vi "Controle_Manip_Main_GUI_WorkingBackup_211222.vi"() -> ()   [LabVIEW 2019] (continued)
                                frame #0 {
                                n1997 = property on="CCD 2D Image Main" class="IntGraph (strict)"("Visible"=FALSE) -> ()  [unwired: 2 in, 2 out]
                                n1998 = property on="CCD 1D Spectrum Main" class="XYGraph (strict)"("Visible"=TRUE) -> ()  [unwired: 2 in, 2 out]
                                }
                                frame #1 {
                                n1999 = local read "Wavelength calibration"() -> (w2451:dbl[])
                                n2000 = local read "CCD ROI"() -> (w2447:T20)
                                n2001 = Divide(x=1239.842, y=w2451) -> (x/y=w2449:dbl[])
                                n2002 = call "PrepareData4Graph.vi"("Wavelength nm"=w2449, "DataLF"=w2454, "CCD ROI"=w2447, "AcqMode"=w2452, "Data type"=T30."Spectre") -> ("Spectrum"=w2453:cluster{"Array 2":dbl[], "Array":dbl[]}, "PLInt out"=w2446:dbl[])  [unwired: 2 in, 2 out]
                                n2003 = local write "CCD 1D Spectrum Main"(w2453) -> ()
                                n2004 = local write "BackgroundSpec"(w2446) -> ()
                                }
                                frame #2 {
                                n2005 = local read "BackgroundSpec"() -> (w2455:dbl[])
                                n2006 = call-poly <vilib>:"Mean.vi"("X"=w2455) -> ("mean"=w2457:dbl)  [unwired: 1 out]
                                n2007 = Negate(x=w2457) -> (-x=w2456:dbl)
                                n2008 = property on="CCD 1D Spectrum Main" class="XYGraph (strict)"("YScale.Offset"=w2456) -> ()  [unwired: 2 in, 2 out]
                                }
                                frame #3 {
                                n2009 = local write "Background taken?"(TRUE ("Background taken?")) -> ()
                                n2010 = property on="Background substract" class="Enum (strict)"("Value"=enum16{"None", "Shutter"}."None" ("Background substract")) -> ()  [unwired: 2 in, 2 out]
                                }
                                }
                                }
                                frame "Image" {
                                n2011 = stacked-sequence {
                                tunnel: w2461 -> [_ w2469]
                                tunnel: w2460 -> [_ w2467]
                                frame #0 {
                                n2012 = property on="CCD 1D Spectrum Main" class="XYGraph (strict)"("Visible"=FALSE) -> ()  [unwired: 2 in, 2 out]
                                n2013 = property on="CCD 2D Image Main" class="IntGraph (strict)"("Visible"=TRUE) -> ()  [unwired: 2 in, 2 out]
                                }
                                frame #1 {
                                n2014 = local read "Wavelength calibration"() -> (w2468:dbl[])
                                n2015 = local read "CCD ROI"() -> (w2464:T20)
                                n2016 = call "PrepareData4Graph.vi"("Wavelength nm"=w2468, "DataLF"=w2469, "CCD ROI"=w2464, "AcqMode"=w2467, "Data type"=T30."Spectre") -> ("Intensity Graph"=w2466:dbl[][])  [unwired: 2 in, 3 out]
                                n2017 = local write "CCD 2D Image Main"(w2466) -> ()
                                }
                                }
                                }
                                }
                              }
                              frame True {
                              }
                            }
                          }
                          frame #1 {
                            w2494 = 1 ("Active X Scale")
                            w2495 = 0
                            # "prep axes for graphs (a nightmare in LabVIEW to not display 1...N but rather Volts or um)"
                            n2018 = local read "Scan X Res. (V)"() -> (w2499:dbl)
                            n2019 = local read "Scan X Tot. Length (V)"() -> (w2497:dbl)
                            n2020 = local read "Scan X Res. (V)"() -> (w2528:dbl)
                            n2021 = local read "Scan X Center (V)"() -> (w2496:dbl)
                            n2022 = local read "Scan X Center (V)"() -> (w2530:dbl)
                            n2023 = local read "Scan Y Center (V)"() -> (w2522:dbl)
                            n2024 = local read "Scan Y Res. (V)"() -> (w2521:dbl)
                            n2025 = local read "Scan Y Tot. Length"() -> (w2524:dbl)
                            n2026 = local read "Scan X Tot. Length (V)"() -> (w2529:dbl)
                            n2027 = local read "V2um"() -> (w2498:dbl)
                            n2028 = call "V2um.vi"("Numeric"=w2499, "V2um"=w2498) -> ("x*y"=w2503:dbl)
                            n2029 = call "V2um.vi"("Numeric"=w2497, "V2um"=w2498) -> ("x*y"=w2500:dbl)
                            n2030 = call "V2um.vi"("Numeric"=w2496, "V2um"=w2498) -> ("x*y"=w2504:dbl)
                            n2031 = Divide(x=w2500, y=w2503) -> (x/y=w2501:dbl)
                            n2032 = local read "Scan Y Res. (V)"() -> (w2510:dbl)
                            n2033 = Divide(x=w2524, y=w2521) -> (x/y=w2525:dbl)
                            n2034 = Increment(x=w2525) -> (x+1=w2523:dbl)
                            n2035 = Increment(x=w2501) -> (x+1=w2502:dbl)
                            n2036 = call "AxXYGraph.vi"("dx"=w2503, "N"=w2502, "x0"=w2504) -> ("Multiplier"=w2493:dbl, "Offset"=w2492:dbl)
                            n2037 = local read "Scan Y Tot. Length"() -> (w2512:dbl)
                            n2038 = Divide(x=w2529, y=w2528) -> (x/y=w2527:dbl)
                            n2039 = local read "Scan Y Center (V)"() -> (w2513:dbl)
                            n2040 = call "AxXYGraph.vi"("dx"=w2521, "N"=w2523, "x0"=w2522) -> ("Multiplier"=w2520:dbl, "Offset"=w2519:dbl)
                            n2041 = Increment(x=w2527) -> (x+1=w2526:dbl)
                            n2042 = call "AxXYGraph.vi"("dx"=w2528, "N"=w2526, "x0"=w2530) -> ("Multiplier"=w2517:dbl, "Offset"=w2518:dbl)
                            n2043 = local read "BackgroundSpec"() -> (w2516:dbl[])
                            n2044 = local read "V2um"() -> (w2511:dbl)
                            n2045 = call "V2um.vi"("Numeric"=w2510, "V2um"=w2511) -> ("x*y"=w2506:dbl)
                            n2046 = call "V2um.vi"("Numeric"=w2512, "V2um"=w2511) -> ("x*y"=w2509:dbl)
                            n2047 = call "V2um.vi"("Numeric"=w2513, "V2um"=w2511) -> ("x*y"=w2505:dbl)
                            n2048 = Divide(x=w2509, y=w2506) -> (x/y=w2508:dbl)
                            n2049 = Increment(x=w2508) -> (x+1=w2507:dbl)
                            n2050 = call "AxXYGraph.vi"("dx"=w2506, "N"=w2507, "x0"=w2505) -> ("Multiplier"=w2491:dbl, "Offset"=w2490:dbl)
                            n2051 = call-poly <vilib>:"Mean.vi"("X"=w2516) -> ("mean"=w2515:dbl)  [unwired: 1 out]
                            n2052 = property on="XY Intensity Map" class="IntGraph (strict)"("ActXScl"=w2495, "XScale.Multiplier"=w2517, "XScale.Offset"=w2518, "ActYScl"=w2495, "YScale.Multiplier"=w2520, "YScale.Offset"=w2519) -> ()  [unwired: 2 in, 2 out]
                            n2053 = property on="XY Intensity Map" class="IntGraph (strict)"("ActXScl"=w2494, "XScale.Multiplier"=w2493, "XScale.Offset"=w2492, "ActYScl"=w2494, "YScale.Multiplier"=w2491, "YScale.Offset"=w2490) -> ()  [unwired: 2 in, 2 out]
                            n2054 = Negate(x=w2515) -> (-x=w2514:dbl)
                            n2055 = property on="CCD 1D Spectrum XY Map" class="XYGraph (strict)"("YScale.Offset"=w2514) -> ()  [unwired: 2 in, 2 out]
                          }
                          frame #2 {
                            w2550 = 1 ("Active Y Scale")
                            w2560 = FALSE
                            w2561 = TRUE ("Visible")
                            # "nightmare part II"
                            n2056 = local read "Scan X Res. (V)"() -> (w2538:dbl)
                            n2057 = local read "Scan Y Center (V)"() -> (w2555:dbl)
                            n2058 = local read "Scan X Center (V)"() -> (w2556:dbl)
                            n2059 = local read "Scanning Mode"() -> (w2565:T21)
                            n2060 = local read "Scan Y Res. (V)"() -> (w2539:dbl)
                            n2061 = property on="Save XY Map" class="Bool (strict)"("Visible"=w2560) -> ()  [unwired: 2 in, 2 out]
                            n2062 = local read "Scan Fast Axis"() -> (w2566:enum16{"Y", "X"})
                            n2063 = property on="Acquire XY Map" class="Bool (strict)"("Visible"=w2560) -> ()  [unwired: 2 in, 2 out]
                            n2064 = local read "Scan XY Map Params"() -> (w2568:refnum<vi>[])
                            n2065 = control-ref of="MasterPause"() -> (w2535:refnum<vi>)
                            n2066 = local read "Scan X Tot. Length (V)"() -> (w2553:dbl)
                            n2067 = local read "Scan Y Tot. Length"() -> (w2554:dbl)
                            n2068 = property on="CCD 1D Spectrum Main Energy Scale" class="XYGraph (strict)"() -> ("XScale.MarkerVals[]"=w2559:dbl[], "XScale.Maximum"=w2558:dbl, "XScale.Minimum"=w2557:dbl)  [unwired: 2 in, 2 out]
                            n2069 = property class="Bool (strict)"(reference=w2535, "Visible"=TRUE) -> ()  [unwired: 1 in, 2 out]
                            n2070 = property on="Experiment Graph Controls" class="TabCtl (strict)"("Value"=T25."XY Intensity Map" ("Experiment Graph Controls")) -> ()  [unwired: 2 in, 2 out]
                            n2071 = call "Enable&Disable_Controls.vi"("Enum"=enum16{"Enabled", "Disabled", "Disabled&Grayed"}."Disabled&Grayed", "References"=w2568) -> ()  [unwired: 1 in]
                            n2072 = Bundle("Scan Fast Axis"=w2566, "Scanning Mode"=w2565, "Scan X Center (V)"=w2556, "Scan X Res. (V)"=w2538, "Scan X Tot. Length (V)"=w2553, "Scan Y Center (V)"=w2555, "Scan Y Res. (V)"=w2539, "Scan Y Tot. Length"=w2554) -> (→"Params XY Map SubVI":T23)  [unwired: 1 in]
                            n2073 = control-ref of="MasterStop"() -> (w2532:refnum<vi>)
                            n2074 = property on="Scan Main Progess Bar" class="Slide (strict)"("Visible"=TRUE, "Value"=u8 0 ("Scan XY Map Progess Bar")) -> ()  [unwired: 2 in, 2 out]
                            n2075 = property on="CCD 1D XY Map Spectrum Main Energy Scale" class="XYGraph (strict)"("XScale.MarkerVals[]"=w2559, "XScale.Maximum"=w2558, "XScale.Minimum"=w2557, "XScale.UniformMarker"=TRUE ("X Scale.Uniform Marker Spacing?")) -> ()  [unwired: 2 in, 2 out]
                            n2076 = local read "V2um"() -> (w2537:dbl)
                            n2077 = property class="Bool (strict)"(reference=w2532, "Visible"=TRUE) -> ()  [unwired: 1 in, 2 out]
                            n2078 = call "AxxXY.vi"("Y Tot"=w2554, "X Tot"=w2553, "Y Res"=w2539, "Y Center"=w2555, "X Res"=w2539, "X Center"=w2556) -> ("YMIN"=w2541:dbl, "YMAX"=w2540:dbl, "XMIN"=w2542:dbl, "XMAX"=w2543:dbl)
                            n2079 = call "V2um.vi"("Numeric"=w2542, "V2um"=w2537) -> ("x*y"=w2548:dbl)
                            n2080 = call "V2um.vi"("Numeric"=w2543, "V2um"=w2537) -> ("x*y"=w2549:dbl)
                            n2081 = call "V2um.vi"("Numeric"=w2541, "V2um"=w2537) -> ("x*y"=w2547:dbl)
                            n2082 = call "V2um.vi"("Numeric"=w2540, "V2um"=w2537) -> ("x*y"=w2546:dbl)
                            n2083 = call "V2um.vi"("Numeric"=w2539, "V2um"=w2537) -> ("x*y"=w2545:dbl)
                            n2084 = call "V2um.vi"("Numeric"=w2538, "V2um"=w2537) -> ("x*y"=w2544:dbl)
                            n2085 = property on="Elapsed (s)" class="DigNum (strict)"("Visible"=w2561) -> ()  [unwired: 2 in, 2 out]
                            n2086 = property on="Expected (s)" class="DigNum (strict)"("Visible"=w2561) -> ()  [unwired: 2 in, 2 out]
                            n2087 = property on="XY Intensity Map" class="IntGraph (strict)"("ActYScl"=0 ("Active Y Scale"), "ActXScl"=0 ("Active X Scale"), "XScale.Maximum"=w2543, "XScale.Minimum"=w2542, "YScale.Minimum"=w2541, "YScale.Maximum"=w2540, "YScale.Increment"=w2539, "XScale.Increment"=w2538) -> ()  [unwired: 2 in, 2 out]
                            n2088 = property on="XY Intensity Map" class="IntGraph (strict)"("ActYScl"=w2550, "ActXScl"=w2550, "XScale.Maximum"=w2549, "XScale.Minimum"=w2548, "YScale.Minimum"=w2547, "YScale.Maximum"=w2546, "YScale.Increment"=w2545, "XScale.Increment"=w2544) -> ()  [unwired: 2 in, 2 out]
                          }
                          frame #3 {
                            w2569 = 0 ("Active X Scale")
                            n2089 = property on="XY Intensity Map" class="IntGraph (strict)"("ActXScl"=w2569, "ActYScl"=w2569) -> ()  [unwired: 2 in, 2 out]
                          }
                          frame #4 {
                            n2090 = local read "Excitation Wavelength (nm)"() -> (w2579:dbl)
                            n2091 = local read "FSM Y Task"() -> (w2590:refnum<k21>)
                            n2092 = local read "FSM X Task"() -> (w2591:refnum<k21>)
                            n2093 = local read "Photodiode handle out"() -> (w2580:refnum<visa-resource-name>)
                            n2094 = local read "LightField Automation out"() -> (w2582:refnum<class "LightField Automation.lvclass">)
                            n2095 = local read "Photodiode error out"() -> (w2578:errorcluster)
                            n2096 = local read "Excitation Wavelength (nm)"() -> (w2586:dbl)
                            n2097 = local read "LightField Automation error out"() -> (w2581:errorcluster)
                            n2098 = local read "KCube Shutter On?"() -> (w2583:bool)
                            n2099 = local read "BackgroundSpec"() -> (w2572:dbl[])
                            n2100 = local read "Accumulations"() -> (w2587:dbl)
                            n2101 = local read "Acq Time (ms)"() -> (w2588:dbl)
                            n2102 = local read "Acq Mode"() -> (w2585:T3)
                            n2103 = local read "CCD ROI"() -> (w2584:T20)
                            n2104 = Bundle("LightField Automation out"=w2582, "LightField Automation error out"=w2581, "FSM X Task"=w2591, "FSM Y Task"=w2590) -> (→"Scan XY Map Handles":T12)  [unwired: 1 in]
                            n2105 = call <instrlib>:"TLPM Set Wavelength.vi"("error in (no error)"=w2578, "Wavelength (0.0)"=w2579, "instrument handle"=w2580) -> ("error out"=w2577:errorcluster, "instrument handle out"=w2576:refnum<visa-resource-name>)  [unwired: 7 in]
                            n2106 = call <instrlib>:"TLPM Measure Power.vi"("error in (no error)"=w2577, "instrument handle"=w2576) -> ("error out"=w2574:errorcluster, "Power"=w2573:dbl, "instrument handle out"=w2575:refnum<visa-resource-name>)  [unwired: 7 in]
                            n2107 = local write "Photodiode handle out"(w2575) -> ()
                            n2108 = local write "Photodiode error out"(w2574) -> ()
                            n2109 = local write "Excitation Power (uW)"(w2573) -> ()
                            n2110 = control-ref of="Display Mode"() -> (w2571:refnum<vi>)
                            n2111 = Bundle("Acq Time (ms)"=w2588, "Accumulations"=w2587, "Excitation Wavelength (nm)"=w2586, "Acq Mode"=w2585, "CCD ROI"=w2584, "KCube Shutter On?"=w2583, "Power"=w2573, "BackgroundSpec"=w2572, "Display Mode"=w2571) -> (→"Scan XY Map Exp Params SubVI":T7)  [unwired: 1 in]
                            n2112 = case shown="True" w2583 {
                              selector: w2583 -> [_ w2592]
                              frame False {
                              }
                              frame True {
                                n2113 = control-ref of="Shutter Ctrls"() -> (w2595:refnum<vi>)
                                n2114 = property class="Ring (strict)"(reference=w2595) -> ("Value"=w2596:u16)  [unwired: 1 in, 2 out]
                                n2115 = control-ref of="KCube Shutter Device Reference"() -> (w2594:refnum<vi>)
                                n2116 = Equal?(x=w2596, y=u16 0) -> (x = y?=w2597:bool)
                                n2117 = case shown="True" w2597 {
                                tunnel: w2594 -> [_ w2600]
                                tunnel: w2595 -> [_ w2599]
                                tunnel: w2592 -> [_ w2598]
                                frame False {
                                }
                                frame True {
                                n2118 = call "Shutter.vi"("KCube Shutter Device Reference 2"=w2600, "Shutter Ctrls 2"=w2599, "Shutter on?"=w2598) -> ()
                                }
                                }
                              }
                            }
                          }
                          frame #5 {
                            n2119 = local read "Scan XY Map Exp Params SubVI"() -> (w2603:T7)
                            n2120 = local read "Scan XY Map References"() -> (w2604:T9)
                            n2121 = local read "Params XY Map SubVI"() -> (w2608:T23)
                            n2122 = local read "Scan XY Map Handles"() -> (w2607:T12)
                            n2123 = call "ScanFSM_v2.vi"("Scan XY Map References"=w2604, "Scan XY Map Handles"=w2607, "Params XY Map SubVI"=w2608, "Scan XY Map Exp Params SubVI"=w2603) -> ("Handles Out"=w2605:T36, "Data"=w2606:i32[][], "XYPos Indices"=w2602:i32[][], "XYPositions"=→"XYPositions":dbl[][])  [unwired: 12 in]
                            n2124 = local write "Scan XY Map Handles"(w2605) -> ()
                            n2125 = local write "XYMap Data"(w2606) -> ()
                            n2126 = local write "XYPos Indices"(w2602) -> ()
                          }
                          frame #6 {
                            n2127 = local read "Scan XY Map Handles"() -> (w2614:T12)
                            n2128 = local read "Scan Y Center (V)"() -> (w2609:dbl)
                            n2129 = local read "Scan X Center (V)"() -> (w2611:dbl)
                            n2130 = local read "KCube Shutter On?"() -> (w2616:bool)
                            n2131 = control-ref of="Shutter Ctrls"() -> (w2618:refnum<vi>)
                            n2132 = local read "FSM X Task"() -> (w2615:refnum<k21>)
                            n2133 = local read "FSM Y Task"() -> (w2610:refnum<k21>)
                            n2134 = control-ref of="KCube Shutter Device Reference"() -> (w2617:refnum<vi>)
                            n2135 = call "Shutter.vi"("KCube Shutter Device Reference 2"=w2617, "Shutter Ctrls 2"=w2618, "Shutter on?"=w2616) -> ()
                            n2136 = call "FSMGoTo.vi"("Target Value (V)"=w2611, "FSM Task"=w2615) -> ()  [unwired: 1 out]
                            n2137 = call "FSMGoTo.vi"("Target Value (V)"=w2609, "FSM Task"=w2610) -> ()  [unwired: 1 out]
                            n2138 = local write "Scan X Readout (V)"(w2611) -> ()
                            n2139 = Unbundle By Name(w2614) -> ("LightField Automation out"=w2613:refnum<class "LightField Automation.lvclass">, "LightField Automation error out"=w2612:errorcluster)
                            n2140 = property on="XY Intensity Map" class="IntGraph (strict)"("Cursor.Cursor X"=w2611) -> ()  [unwired: 2 in, 2 out]
                            n2141 = local write "Scan Y Readout (V)"(w2609) -> ()
                            n2142 = property on="XY Intensity Map" class="IntGraph (strict)"("Cursor.Cursor Y"=w2609) -> ()  [unwired: 2 in, 2 out]
                            n2143 = local write "LightField Automation error out"(w2612) -> ()
                            n2144 = local write "LightField Automation out"(w2613) -> ()
                          }
                          frame #7 {
                            w2619 = T29."Disabled and Grayed Out" ("Disabled")
                            w2632 = FALSE ("Visible")
                            n2145 = local read "Scan XY Map Params"() -> (w2636:refnum<vi>[])
                            n2146 = local read "Auto< ?"() -> (w2625:bool)
                            n2147 = local write "Acquire XY Map"(FALSE ("Acquire XY Map")) -> ()
                            n2148 = local write "Save XY Map"(FALSE ("Acquire XY Map")) -> ()
                            n2149 = case shown="True" w2625 {
                              tunnel: [TRUE FALSE] -> w2624
                              frame False {
                              }
                              frame True {
                              }
                            }
                            n2150 = call "Enable&Disable_Controls.vi"("Enum"=enum16{"Enabled", "Disabled", "Disabled&Grayed"}."Enabled", "References"=w2636) -> ()  [unwired: 1 in]
                            n2151 = property on="Acquire XY Map" class="Bool (strict)"("Visible"=TRUE, "Value"=FALSE ("Acquire XY Map")) -> ()  [unwired: 2 in, 2 out]
                            n2152 = local write "ExportMapPosition?"(TRUE ("ExportMapPosition?")) -> ()
                            n2153 = disable-structure shown="Disabled" {
                              disable-tunnel: w2632 -> [w2639 _]
                              frame Disabled {
                                n2154 = property on="Scan Main Progess Bar" class="Slide (strict)"("Visible"=w2639) -> ()  [unwired: 2 in, 2 out]
                              }
                              frame Enabled {
                              }
                            }
                            n2155 = property on="Save XY Map" class="Bool (strict)"("Visible"=w2624) -> ()  [unwired: 2 in, 2 out]
                            n2156 = property on="Elapsed (s)" class="DigNum (strict)"("Visible"=w2632) -> ("Value"=w2622:dbl)  [unwired: 2 in, 2 out]
                            n2157 = control-ref of="MasterStop"() -> (w2627:refnum<vi>)
                            n2158 = control-ref of="Scanning Mode"() -> (w2621:refnum<vi>)
                            n2159 = control-ref of="Scan Fast Axis"() -> (w2620:refnum<vi>)
                            n2160 = control-ref of="MasterPause"() -> (w2628:refnum<vi>)
                            n2161 = local write "Scan Main Progess Bar"(u8 0 ("Scan Main Progess Bar")) -> ()
                            n2162 = control-ref of="ExperimentStopped?"() -> (w2626:refnum<vi>)
                            n2163 = call "CheckStopAndReset.vi"("ExperimentStopped?"=w2626, "MasterStop"=w2627, "MasterPause"=w2628) -> ()
                            n2164 = property on="Expected (s)" class="DigNum (strict)"("Value"=w2622) -> ()  [unwired: 2 in, 2 out]
                            n2165 = property class="Enum (strict)"(reference=w2620, "DisabledEnum"=w2619) -> ()  [unwired: 1 in, 2 out]
                            n2166 = property class="Enum (strict)"(reference=w2621, "DisabledEnum"=w2619) -> ()  [unwired: 1 in, 2 out]
                          }
                        }
                      }
                      frame "Acquire Contrast test array of references" {
                        n2167 = stacked-sequence {
                          frame #0 {
                            w2642 = FALSE
                            w2643 = TRUE
                            w2651 = FALSE ("Acq Cont")
                            w2648 = FALSE ("Acq Cont")
                            n2168 = property on="CCD 1D Spectrum Main" class="XYGraph (strict)"() -> ("XScale.Maximum"=w2647:dbl, "XScale.Minimum"=w2646:dbl, "YScale.Minimum"=w2645:dbl, "YScale.Maximum"=w2644:dbl)  [unwired: 2 in, 2 out]
                            n2169 = property on="Acquire Contrast" class="Bool (strict)"("Visible"=w2642) -> ()  [unwired: 2 in, 2 out]
                            n2170 = property on="Save Contrast" class="Bool (strict)"("Visible"=w2642) -> ()  [unwired: 2 in, 2 out]
                            n2171 = property on="Scan Linear Stage Progess Bar" class="Slide (strict)"("Visible"=TRUE, "Value"=u8 0 ("Scan Linear Stage Progess Bar")) -> ()  [unwired: 2 in, 2 out]
                            n2172 = property on="Pause Contrast" class="Bool (strict)"("Visible"=w2643) -> ()  [unwired: 2 in, 2 out]
                            n2173 = property on="Stop Contrast" class="Bool (strict)"("Visible"=w2643) -> ()  [unwired: 2 in, 2 out]
                            n2174 = property on="Contrast 1D Spectrum" class="XYGraph (strict)"("XScale.Maximum"=w2647, "XScale.Minimum"=w2646, "YScale.Minimum"=w2645, "YScale.Maximum"=w2644) -> ()  [unwired: 2 in, 2 out]
                            n2175 = local read "Scan Contrast Ctrls"() -> (w2652:refnum<vi>[])
                            n2176 = property on="Experiment Graph Controls" class="TabCtl (strict)"("Value"=T25."Contrast" ("Experiment Graph Controls")) -> ()  [unwired: 2 in, 2 out]
                            n2177 = property on="Scan Linear Stage Progess Bar" class="Slide (strict)"("Visible"=TRUE) -> ()  [unwired: 2 in, 2 out]
                            n2178 = call "Enable&Disable_Controls.vi"("Enum"=enum16{"Enabled", "Disabled", "Disabled&Grayed"}."Disabled&Grayed", "References"=w2652) -> ()  [unwired: 1 in]
                            n2179 = local write "Acquire Contrast"(w2648) -> ()
                            n2180 = local write "Save Contrast"(w2648) -> ()
                            n2181 = local write "Pause Contrast"(w2651) -> ()
                            n2182 = local write "Stop Contrast"(w2651) -> ()
                          }
                          frame #1 {
                            n2183 = local read "ESP 301 COM Port"() -> (w2667:refnum<visa-resource-name>)
                            n2184 = local read "Photodiode handle out"() -> (w2665:refnum<visa-resource-name>)
                            n2185 = local read "Photodiode error out"() -> (w2664:errorcluster)
                            n2186 = local read "LightField Automation error out"() -> (w2654:errorcluster)
                            n2187 = local read "LinTFine End Pos (usteps)"() -> (w2671:dbl)
                            n2188 = local read "LinTFines Step Pos (usteps)"() -> (w2672:dbl)
                            n2189 = local read "LinTFine Start Pos (usteps)"() -> (w2673:dbl)
                            n2190 = local read "PZC200 Instrument Channel"() -> (w2669:string)
                            n2191 = local read "LinT End pos (mm)"() -> (w2674:dbl)
                            n2192 = local read "LightField Automation out"() -> (w2655:refnum<class "LightField Automation.lvclass">)
                            n2193 = local read "LinT Step Pos (mm)"() -> (w2675:dbl)
                            n2194 = local read "LinT Start Pos (mm)"() -> (w2676:dbl)
                            n2195 = local read "ESP 301 Error"() -> (w2666:errorcluster)
                            n2196 = local read "PZC Error"() -> (w2668:errorcluster)
                            n2197 = Bundle("LinT Start Pos (mm)"=w2676, "LinT Step Pos (mm)"=w2675, "LinT End pos (mm)"=w2674, "LinTFine Start Pos (usteps)"=w2673, "LinTFines Step Pos (usteps)"=w2672, "LinTFine End Pos (usteps)"=w2671) -> (w2670:T27)  [unwired: 1 in]
                            n2198 = local read "Excitation Wavelength (nm)"() -> (w2660:dbl)
                            n2199 = Bundle("LightField Automation out"=w2655, "LightField Automation error out"=w2654, "PZC200 Instrument Channel"=w2669, "PZC Error"=w2668, "ESP 301 COM Port"=w2667, "ESP 301 Error"=w2666, "Photodiode handle out"=w2665, "Photodiode error out"=w2664) -> (w2663:T13)  [unwired: 1 in]
                            n2200 = local read "Exposure Time (ms)"() -> (w2662:dbl)
                            n2201 = local read "KCube Shutter On?"() -> (w2656:bool)
                            n2202 = local read "Accumulations"() -> (w2661:dbl)
                            n2203 = local read "Acq Mode"() -> (w2659:T3)
                            n2204 = local read "CCD ROI"() -> (w2658:T20)
                            n2205 = local write "Scan Translation Params"(w2670) -> ()
                            n2206 = local write "Constrast Handles"(w2663) -> ()
                            n2207 = Bundle("Exposure Time (ms)"=w2662, "Accumulations"=w2661, "Excitation Wavelength (nm)"=w2660, "Acq Mode"=w2659, "CCD ROI"=w2658, "KCube Shutter On?"=w2656) -> (w2657:T24)  [unwired: 1 in]
                            n2208 = local write "Scan Translation Exp Params"(w2657) -> ()
                          }
                          frame #2 {
                            n2209 = local read "Scan Translation Exp Params"() -> (w2681:T24)
                            n2210 = local read "Contrast References"() -> (w2680:T14)
                            n2211 = local read "Scan Translation Params"() -> (w2682:T27)
                            n2212 = local read "Constrast Handles"() -> (w2683:T13)
                            n2213 = call "FineContrast_v3.0.vi"("Contrast References"=w2680, "Constrast Handles"=w2683, "Scan Translation Exp Params"=w2681, "Scan Translation Params"=w2682) -> ("Constrast Handles Out"=w2679:T37)  [unwired: 2 out]
                            n2214 = Unbundle By Name(w2679) -> ("LightField Automation out"=w2678:refnum<class "LightField Automation.lvclass">, "error out"=w2677:errorcluster)
                            n2215 = local write "Constrast Handles"(w2679) -> ()
                            n2216 = local write "LightField Automation error out"(w2677) -> ()
                            n2217 = local write "LightField Automation out"(w2678) -> ()
                          }
                          frame #3 {
                            w2685 = TRUE
                            w2684 = FALSE
                            w2689 = FALSE ("Acq Cont")
                            w2686 = FALSE ("Acq Cont")
                            n2218 = property on="Scan Linear Stage Progess Bar" class="Slide (strict)"("Visible"=FALSE, "Value"=u8 0 ("Scan Linear Stage Progess Bar")) -> ()  [unwired: 2 in, 2 out]
                            n2219 = property on="Acquire Contrast" class="Bool (strict)"("Visible"=w2685) -> ()  [unwired: 2 in, 2 out]
                            n2220 = property on="Save Contrast" class="Bool (strict)"("Visible"=w2685) -> ()  [unwired: 2 in, 2 out]
                            n2221 = property on="Pause Contrast" class="Bool (strict)"("Visible"=w2684) -> ()  [unwired: 2 in, 2 out]
                            n2222 = property on="Stop Contrast" class="Bool (strict)"("Visible"=w2684) -> ()  [unwired: 2 in, 2 out]
                            n2223 = local read "Scan Contrast Ctrls"() -> (w2690:refnum<vi>[])
                            n2224 = local write "Acquire Michelson"(w2686) -> ()
                            n2225 = local write "Acquire Contrast"(w2686) -> ()
                            n2226 = local write "Save Michelson"(w2686) -> ()
                            n2227 = local write "Pause Michelson"(w2689) -> ()
                            n2228 = local write "Stop Michelson"(w2689) -> ()
                            n2229 = call "Enable&Disable_Controls.vi"("Enum"=enum16{"Enabled", "Disabled", "Disabled&Grayed"}."Enabled", "References"=w2690) -> ()  [unwired: 1 in]
                          }
                        }
                      }
                      frame "Acquire Contrast EVERYTHING OK" {
                        n2230 = stacked-sequence {
                          tunnel: [_ w2707 _] -> _
                          frame #0 {
                            w2699 = FALSE
                            w2702 = TRUE
                            n2231 = property on="Stop Contrast" class="Bool (strict)"("Visible"=w2702) -> ()  [unwired: 2 in, 2 out]
                            n2232 = property on="Pause Contrast" class="Bool (strict)"("Visible"=w2702) -> ()  [unwired: 2 in, 2 out]
                            n2233 = property on="Experiment Graph Controls" class="TabCtl (strict)"("Value"=T25."Contrast" ("Experiment Graph Controls")) -> ()  [unwired: 2 in, 2 out]
                            n2234 = local read "Scan Contrast Ctrls"() -> (w2700:refnum<vi>[])
                            n2235 = property on="Save Contrast" class="Bool (strict)"("Visible"=w2699) -> ()  [unwired: 2 in, 2 out]
                            n2236 = property on="Acquire Contrast" class="Bool (strict)"("Visible"=w2699) -> ()  [unwired: 2 in, 2 out]
                            n2237 = call "Enable&Disable_Controls.vi"("Enum"=enum16{"Enabled", "Disabled", "Disabled&Grayed"}."Disabled&Grayed", "References"=w2700) -> ()  [unwired: 1 in]
                            n2238 = property on="CCD 1D Spectrum Main" class="XYGraph (strict)"() -> ("XScale.Maximum"=w2698:dbl, "XScale.Minimum"=w2697:dbl, "YScale.Minimum"=w2696:dbl, "YScale.Maximum"=w2695:dbl)  [unwired: 2 in, 2 out]
                            n2239 = property on="Scan Linear Stage Progess Bar" class="Slide (strict)"("Visible"=TRUE, "Value"=u8 0 ("Scan Linear Stage Progess Bar")) -> ()  [unwired: 2 in, 2 out]
                            n2240 = property on="Contrast 1D Spectrum" class="XYGraph (strict)"("XScale.Maximum"=w2698, "XScale.Minimum"=w2697, "YScale.Minimum"=w2696, "YScale.Maximum"=w2695) -> ()  [unwired: 2 in, 2 out]
                          }
                          frame #1 {
                            n2241 = local read "Excitation Wavelength (nm)"() -> (w2711:dbl)
                            n2242 = local read "LinTFines Step Pos (usteps)"() -> (w2715:dbl)
                            n2243 = local read "LinTFine Start Pos (usteps)"() -> (w2717:dbl)
                            n2244 = local read "LinTFine End Pos (usteps)"() -> (w2716:dbl)
                            n2245 = local read "Exposure Time (ms)"() -> (w2713:dbl)
                            n2246 = local read "LightField Automation error out"() -> (w2703:errorcluster)
                            n2247 = local read "Acq Mode"() -> (w2712:T3)
                            n2248 = local read "CCD ROI"() -> (w2707:T20)
                            n2249 = local read "LightField Automation out"() -> (w2704:refnum<class "LightField Automation.lvclass">)
                            n2250 = control-ref of="KCube Shutter Device Reference"() -> (w2719:refnum<vi>)
                            n2251 = control-ref of="PZC Position Readout (usteps)"() -> (w2726:refnum<vi>)
                            n2252 = control-ref of="Scan Linear Stage Progess Bar"() -> (w2725:refnum<vi>)
                            n2253 = local read "PZC200 Instrument Channel"() -> (w2718:string)
                            n2254 = control-ref of="Contrast Oscillations"() -> (w2723:refnum<vi>)
                            n2255 = control-ref of="Pause Contrast"() -> (w2724:refnum<vi>)
                            n2256 = control-ref of="Contrast 1D Spectrum"() -> (w2722:refnum<vi>)
                            n2257 = Open VI Reference(type specifier VI Refnum (for type only)=refnum<vi> refnum ("application reference (local)"), vi path=path "D:/Users/manip-thz/Documents/Controle_Manip_2020/subVIs/Scans/FineContrast.vi", options=256) -> (vi reference=w2733:refnum<vi>, error out=w2732:errorcluster)  [unwired: 3 in]
                            n2258 = control-ref of="Stop Contrast"() -> (w2721:refnum<vi>)
                            n2259 = local read "PZC Error"() -> (w2727:errorcluster)
                            n2260 = control-ref of="Shutter Ctrls"() -> (w2720:refnum<vi>)
                            n2261 = call-by-ref "Wait On Asynchronous Call"(reference=w2733, error in=w2732) -> (reference out=w2729:refnum<vi>, error out=w2728:errorcluster, "LightField Automation out"=w2705:refnum<class "LightField Automation.lvclass">, "PZC200 Instrument Channel 2"=w2731:string, "PZC Error 2"=w2730:errorcluster, "PZAPos & InstPow"=w2708:dbl[][], "Spectra vs PZA"=w2714:i32[][], "LightField Automation error  out"=w2706:errorcluster)  [unwired: 22 in]
                            n2262 = local write "PZAPos&Pow"(w2708) -> ()
                            n2263 = Close Reference(reference=w2729, error in (no error)=w2728) -> ()  [unwired: 1 out]
                            n2264 = local write "PZC Error"(w2730) -> ()
                            n2265 = local write "Contrast Array Out"(w2714) -> ()
                            n2266 = local write "PZC200 Instrument Channel"(w2731) -> ()
                            n2267 = local read "Photodiode handle out"() -> (w2709:refnum<visa-resource-name>)
                            n2268 = local read "Photodiode error out"() -> (w2710:errorcluster)
                            n2269 = call-by-ref "Start Asynchronous Call"(reference=w2733, error in=w2732, "LightField Automation"=w2704, "PZC200 Instrument Channel"=w2718, "ExcWL_nm"=w2711, "PZC Error"=w2727, "Acq Time (ms) 2"=w2713, "Acq Mode"=w2712, "CCD ROI"=w2707, "LightField Automation error"=w2703, "Shutter Device Reference"=w2719, "PZC Position Readout (usteps) 2"=w2726, "LinTFine Start"=w2717, "LinTFine End"=w2716, "Shutter Controls"=w2720, "Scan Spectrum Progess Bar 2"=w2725, "Stop Contrast 2"=w2721, "Pause Contrast 2"=w2724, "Contrast 1D Spectrum 2"=w2722, "LinTFine Step"=w2715, "Contrast Oscillations 2"=w2723, "Photodiode handle out"=w2709, "Photodiode error out"=w2710) -> ()  [unwired: 1 in, 8 out]
                            n2270 = local write "LightField Automation error out"(w2706) -> ()
                            n2271 = local write "LightField Automation out"(w2705) -> ()
                          }
                          frame #2 {
                            w2740 = FALSE ("Acq Cont")
                            w2737 = FALSE ("Acq Cont")
                            w2741 = TRUE
                            w2744 = FALSE
                            n2272 = property on="Stop Contrast" class="Bool (strict)"("Visible"=w2744) -> ()  [unwired: 2 in, 2 out]
                            n2273 = property on="Pause Contrast" class="Bool (strict)"("Visible"=w2744) -> ()  [unwired: 2 in, 2 out]
                            n2274 = local read "Scan Contrast Ctrls"() -> (w2742:refnum<vi>[])
                            n2275 = property on="Save Contrast" class="Bool (strict)"("Visible"=w2741) -> ()  [unwired: 2 in, 2 out]
                            n2276 = property on="Acquire Contrast" class="Bool (strict)"("Visible"=w2741) -> ()  [unwired: 2 in, 2 out]
                            n2277 = call "Enable&Disable_Controls.vi"("Enum"=enum16{"Enabled", "Disabled", "Disabled&Grayed"}."Enabled", "References"=w2742) -> ()  [unwired: 1 in]
                            n2278 = local write "Acquire Contrast"(w2737) -> ()
                            n2279 = local write "Save Contrast"(w2737) -> ()
                            n2280 = local write "Pause Contrast"(w2740) -> ()
                            n2281 = local write "Stop Contrast"(w2740) -> ()
                            n2282 = property on="Scan Linear Stage Progess Bar" class="Slide (strict)"("Visible"=TRUE, "Value"=u8 0 ("Scan Linear Stage Progess Bar")) -> ()  [unwired: 2 in, 2 out]
                          }
                        }
                      }
                    }
                  }
                }
              }
              frame #1 {
                # "AutoSave?"
                n2283 = local read "ExperimentStopped?"() -> (w2747:bool)
                n2284 = property class="Bool"(reference=w2750) -> ("Label.Text"=w2749:string)  [unwired: 1 in, 2 out]
                n2285 = Not(x=w2747) -> (.not. x?=w2746:bool)
                n2286 = local read "Auto< ?"() -> (w2748:bool)
                n2287 = And(x=w2748, y=w2746) -> (x .and. y?=w2745:bool)
                n2288 = case shown="True" w2745 {
                  tunnel: w2749 -> [_ w2751]
                  frame False {
                  }
                  frame True {
                    n2289 = case shown="\"Acquire XY Map\"" w2751 {
                      frame "Acquire Continuous Spectrum" {
                      }
                      frame "Fast Acq Continuous" {
                      }
                      frame "Acquire Polarisation" {
                        n2290 = property on="Save Polarisation" class="Bool (strict)"("Val(Sgnl)"=TRUE ("Value (Signaling)")) -> ()  [unwired: 2 in, 2 out]
                      }
                      frame "Acquire fPow" {
                        n2291 = property on="Save fPow" class="Bool (strict)"("Val(Sgnl)"=TRUE ("Value (Signaling)")) -> ()  [unwired: 2 in, 2 out]
                      }
                      frame "Acquire XY Map" {
                        n2292 = property on="Save XY Map" class="Bool (strict)"("Val(Sgnl)"=TRUE ("Value (Signaling)")) -> ()  [unwired: 2 in, 2 out]
                      }
                      frame "Acquire Contrast" {
                        n2293 = property on="Save Contrast" class="Bool (strict)"("Val(Sgnl)"=TRUE ("Value (Signaling)")) -> ()  [unwired: 2 in, 2 out]
                      }
                      frame "Acquire Time Trace" {
                        n2294 = property on="Save Spectrum N" class="Bool (strict)"("Val(Sgnl)"=TRUE ("Value (Signaling)")) -> ()  [unwired: 2 in, 2 out]
                      }
                      frame Default {
                      }
                      frame "Acquire Custom Diode Spectrum" {
                        n2295 = property on="Save Custom Diode Spectrum" class="Bool (strict)"("Val(Sgnl)"=TRUE) -> ()  [unwired: 2 in, 2 out]
                      }
                      frame "Acquire PLE" {
                        n2296 = property on="Save PLE" class="Bool (strict)"("Val(Sgnl)"=TRUE ("Value (Signaling)")) -> ()  [unwired: 2 in, 2 out]
                      }
                      frame "Acquire Michelson" {
                        n2297 = property on="Save Michelson" class="Bool (strict)"("Val(Sgnl)"=TRUE ("Value (Signaling)")) -> ()  [unwired: 2 in, 2 out]
                      }
                      frame "Acquire Spectrum" {
                        n2298 = property on="Save Spectrum" class="Bool (strict)"("Val(Sgnl)"=TRUE ("Value (Signaling)")) -> ()  [unwired: 2 in, 2 out]
                      }
                      frame "Fast Acq" {
                      }
                    }
                  }
                }
              }
            }
          }
          event "Doc Cryostat", "Doc LLTF", "Doc ESP 301", "Doc Shutter", "Doc PZC200", "Doc NanoMax", "Doc Attocubes", "Doc LightField", "Doc PicoHarp", "Doc Photodiode", "Doc ESP 300", "Doc FSM": Mouse Down {
            n2299 = event-data() -> ("CtlRef"=w2766:refnum<vi>)  [unwired: 1 in, 7 out]
            n2300 = property class="Bool (strict)"(reference=w2766) -> ("Label.Text"=w2765:string)  [unwired: 1 in, 2 out]
            n2301 = case shown="\"Doc LightField\"" w2765 {
              tunnel: ["\"C:\\Users\\manip\\Documents\\Controle_Manip_2020\\Documentation\\Attocubes\\Positioners\\Manual_FlexPositioners_&_Scanner_v2.2.pdf\"" "\"C:\\Users\\manip\\Documents\\Controle_Manip_2020\\subVIs\\Light Field\\LightField-Users-Manual-Issue-4.5-4411-0125.pdf\"" "\"C:\\Users\\manip\\Documents\\Controle_Manip_2020\\subVIs\\Newport\\NanoPZ-User-Manual-RevA.pdf\"" "\"C:\\Users\\manip\\Documents\\Controle_Manip_2020\\subVIs\\Kinesis\\MAX312D_M-Manual.pdf\"" "\"C:\\Users\\manip\\Documents\\Controle_Manip_2020\\subVIs\\PicoHarp\\Manual.pdf\" " ("command line") "\"C:\\Users\\manip\\Documents\\Controle_Manip_2020\\subVIs\\TLPM\\PM16-121-SpecSheet.pdf\"" "\"C:\\Cryostation\\Help.pdf\"" "\"C:\\Users\\manip\\Desktop\\Photon etc\\PHySpec\\manuals\\LLTF Getting started 1.14.pdf\"" "\"C:\\Newport\\Motion Control\\ESP301\\Doc\\ESP301 - Controller GUI Manual.pdf\"" "\"C:\\Users\\manip\\Documents\\Controle_Manip_2020\\subVIs\\Newport\\Newport ESP300\\ESP300.pdf\"" "\"C:\\Users\\manip\\Documents\\Controle_Manip_2020\\subVIs\\Kinesis\\SH05_M-Manual.pdf\"" "\"C:\\Users\\manip\\Documents\\Controle_Manip_2020\\Documentation\\Misc\\FSM-300UserManual.pdf\""] -> w2761
              frame "Doc Attocubes" {
              }
              frame "Doc LightField" {
              }
              frame "Doc PZC200" {
              }
              frame "Doc NanoMax" {
              }
              frame "Doc PicoHarp" {
              }
              frame "Doc Photodiode" {
              }
              frame "Doc Cryostat", Default {
              }
              frame "Doc LLTF" {
              }
              frame "Doc ESP 301" {
              }
              frame "Doc ESP 300" {
              }
              frame "Doc Shutter" {
              }
              frame "Doc FSM" {
              }
            }
            n2302 = Concatenate Strings("\"C:\\Program Files\\Adobe\\Acrobat DC\\Acrobat\\Acrobat.exe\" " ("command line"), w2761) -> (w2763:string)
            n2303 = call <vilib>:"System Exec.vi"("wait until completion? (T)"=FALSE, "command line"=w2763) -> ()  [unwired: 6 in, 4 out]
          }
          event "PLE Start (nm)", "PLE End (nm)", "PLE Step (nm)": Value Change {
            n2304 = event-data() -> ()  [unwired: 1 in, 6 out]
            n2305 = local read "PLE End (nm)"() -> (w2785:dbl)
            n2306 = local read "PLE Step (nm)"() -> (w2782:dbl)
            n2307 = local read "PLE Start (nm)"() -> (w2784:dbl)
            n2308 = Subtract(x=w2785, y=w2784) -> (x-y=w2783:dbl)
            n2309 = local read "Acq Time (ms)"() -> (w2789:dbl)
            n2310 = Divide(x=w2783, y=w2782) -> (x/y=w2790:dbl)
            n2311 = Add(x=w2789, y=200.0) -> (x+y=w2788:dbl)
            n2312 = Increment(x=w2790) -> (x+1=w2781:dbl)
            "PLE # Pts" <- w2781
            n2313 = Divide(x=w2788, y=1000.0) -> (x/y=w2780:dbl)
            n2314 = Multiply(x=w2781, y=w2780) -> (x*y=w2779:dbl)
            n2315 = control-ref of="Expected (s)"() -> (w2791:refnum<vi>)
            n2316 = property class="DigNum (strict)"(reference=w2791, "Value"=w2779) -> ()  [unwired: 1 in, 2 out]
          }
          event "Display Mode": Value Change {
            n2317 = event-data() -> ("CtlRef"=w2793:refnum<vi>)  [unwired: 1 in, 5 out]
            n2318 = property class="Ring (strict)"(reference=w2793) -> ("Label.Text"=w2792:string)  [unwired: 1 in, 2 out]
            n2319 = case shown="\"Display Mode\"" w2792 {
              frame "False", Default {
              }
              frame "Display Mode" {
                n2320 = local read "Excitation Power (uW)"() -> (w2796:dbl)
                n2321 = local read "BackgroundSpec"() -> (w2797:dbl[])
                n2322 = local read "Acq Time (ms)"() -> (w2795:dbl)
                n2323 = property on="CCD 1D Spectrum Main" class="XYGraph (strict)"() -> ("Value"=w2799:cluster{dbl[], dbl[]})  [unwired: 2 in, 2 out]
                n2324 = local read "Display Mode"() -> (w2800:u16)
                n2325 = Unbundle(w2799) -> (w2798:dbl[])  [unwired: 1 out]
                n2326 = control-ref of="Cnts"() -> (w2794:refnum<vi>)
                n2327 = call "2Cnts.vi"("Array Background"=w2797, "Pow W"=w2796, "AcqTime ms"=w2795, "Cnts Ref"=w2794, "Display Mode"=w2800, "Array"=w2798) -> ()  [unwired: 1 out]
              }
            }
          }
          event "Spectrum Custom Mode": Value Change {
            # "make sure proper input before calibration"
            n2328 = event-data() -> ("NewVal"=w2805:u16)  [unwired: 1 in, 5 out]
            n2329 = case shown="2" w2805 {
              tunnel: [350.0 350.0 350.0 350.0 350.0] -> w2802
              tunnel: [900.0 900.0 900.0 900.0 900.0] -> w2801
              frame 0, Default {
              }
              frame 1 {
              }
              frame 3 {
              }
              frame 2 {
              }
              frame 4 {
              }
            }
            n2330 = control-ref of="Spectrum Start Wavelength (nm)"() -> (w2804:refnum<vi>)
            n2331 = control-ref of="Spectrum End Wavelength (nm)"() -> (w2803:refnum<vi>)
            n2332 = property class="DigNum (strict)"(reference=w2803, "Maximum"=w2801, "Minimum"=w2802) -> ()  [unwired: 1 in, 2 out]
            n2333 = property class="DigNum (strict)"(reference=w2804, "Maximum"=w2801, "Minimum"=w2802) -> ()  [unwired: 1 in, 2 out]
          }
          event Value Change {
            # "APD, CCD Image or binned CCD image"
            n2334 = event-data() -> ()  [unwired: 1 in, 6 out]
            n2335 = local read "Acq Mode"() -> (w2817:T3)
            n2336 = case shown="\"Image\"" w2817 {
              frame "Image" {
                w2819 = TRUE
                w2820 = FALSE
                n2337 = property on="CCD 1D Spectrum XY Map" class="WFGraph (strict)"("Visible"=w2820) -> ()  [unwired: 2 in, 2 out]
                n2338 = property on="CCD 1D Spectrum Main" class="XYGraph (strict)"("Visible"=w2820) -> ()  [unwired: 2 in, 2 out]
                n2339 = property on="Background substract" class="Enum (strict)"("Visible"=w2819) -> ()  [unwired: 2 in, 2 out]
                n2340 = property on="CCD ROI" class="Enum (strict)"("Visible"=w2819) -> ()  [unwired: 2 in, 2 out]
                n2341 = property on="Exit mirror" class="Ring (strict)"("Val(Sgnl)"=u16 4 ("Value (Signaling)")) -> ()  [unwired: 2 in, 2 out]
                n2342 = property on="Accumulations" class="DigNum (strict)"("Visible"=w2819) -> ()  [unwired: 2 in, 2 out]
                n2343 = property on="CCD 2D Image Main" class="IntGraph (strict)"("Visible"=w2819) -> ()  [unwired: 2 in, 2 out]
                n2344 = property on="CCD 2D Image XY Map" class="IntGraph (strict)"("Visible"=w2819) -> ()  [unwired: 2 in, 2 out]
                n2345 = property on="Exposure Time (ms)" class="DigNum (strict)"("Visible"=w2819) -> ()  [unwired: 2 in, 2 out]
              }
              frame "Spectrum" {
                w2823 = FALSE
                w2822 = TRUE
                n2346 = property on="Exit mirror" class="Ring (strict)"("Val(Sgnl)"=u16 4 ("Value (Signaling)")) -> ()  [unwired: 2 in, 2 out]
                n2347 = property on="CCD 2D Image XY Map" class="IntGraph (strict)"("Visible"=w2823) -> ()  [unwired: 2 in, 2 out]
                n2348 = property on="CCD 2D Image Main" class="IntGraph (strict)"("Visible"=w2823) -> ()  [unwired: 2 in, 2 out]
                n2349 = property on="Background substract" class="Enum (strict)"("Visible"=w2822) -> ()  [unwired: 2 in, 2 out]
                n2350 = property on="CCD ROI" class="Enum (strict)"("Visible"=w2822) -> ()  [unwired: 2 in, 2 out]
                n2351 = property on="Accumulations" class="DigNum (strict)"("Visible"=w2822) -> ()  [unwired: 2 in, 2 out]
                n2352 = property on="CCD 1D Spectrum XY Map" class="WFGraph (strict)"("Visible"=w2822) -> ()  [unwired: 2 in, 2 out]
                n2353 = property on="Exposure Time (ms)" class="DigNum (strict)"("Visible"=w2822) -> ()  [unwired: 2 in, 2 out]
                n2354 = property on="CCD 1D Spectrum Main" class="XYGraph (strict)"("Visible"=w2822) -> ()  [unwired: 2 in, 2 out]
              }
              frame "APD 1" {
                w2825 = FALSE
                w2826 = TRUE
                n2355 = property on="CCD 1D Spectrum XY Map" class="WFGraph (strict)"("Visible"=w2826) -> ()  [unwired: 2 in, 2 out]
                n2356 = property on="CCD 1D Spectrum Main" class="XYGraph (strict)"("Visible"=w2826) -> ()  [unwired: 2 in, 2 out]
                n2357 = property on="Exit mirror" class="Ring (strict)"("Val(Sgnl)"=u16 5 ("Value (Signaling)")) -> ()  [unwired: 2 in, 2 out]
                n2358 = property on="Background substract" class="Enum (strict)"("Visible"=w2825) -> ()  [unwired: 2 in, 2 out]
                n2359 = property on="CCD ROI" class="Enum (strict)"("Visible"=w2825) -> ()  [unwired: 2 in, 2 out]
                n2360 = property on="Accumulations" class="DigNum (strict)"("Visible"=w2825) -> ()  [unwired: 2 in, 2 out]
                n2361 = property on="CCD 2D Image Main" class="IntGraph (strict)"("Visible"=w2825) -> ()  [unwired: 2 in, 2 out]
                n2362 = property on="CCD 2D Image XY Map" class="IntGraph (strict)"("Visible"=w2825) -> ()  [unwired: 2 in, 2 out]
                n2363 = property on="Exposure Time (ms)" class="DigNum (strict)"("Visible"=w2825) -> ()  [unwired: 2 in, 2 out]
              }
              frame "APD 2" {
                w2827 = FALSE
                w2828 = TRUE
                n2364 = property on="CCD 1D Spectrum XY Map" class="WFGraph (strict)"("Visible"=w2828) -> ()  [unwired: 2 in, 2 out]
                n2365 = property on="CCD 1D Spectrum Main" class="XYGraph (strict)"("Visible"=w2828) -> ()  [unwired: 2 in, 2 out]
                n2366 = property on="Background substract" class="Enum (strict)"("Visible"=w2827) -> ()  [unwired: 2 in, 2 out]
                n2367 = property on="CCD ROI" class="Enum (strict)"("Visible"=w2827) -> ()  [unwired: 2 in, 2 out]
                n2368 = property on="Accumulations" class="DigNum (strict)"("Visible"=w2827) -> ()  [unwired: 2 in, 2 out]
                n2369 = property on="CCD 2D Image Main" class="IntGraph (strict)"("Visible"=w2827) -> ()  [unwired: 2 in, 2 out]
                n2370 = property on="CCD 2D Image XY Map" class="IntGraph (strict)"("Visible"=w2827) -> ()  [unwired: 2 in, 2 out]
                n2371 = property on="Exposure Time (ms)" class="DigNum (strict)"("Visible"=w2827) -> ()  [unwired: 2 in, 2 out]
              }
              frame "APD 1+2" {
                w2830 = FALSE
                w2831 = TRUE
                n2372 = property on="CCD 1D Spectrum XY Map" class="WFGraph (strict)"("Visible"=w2831) -> ()  [unwired: 2 in, 2 out]
                n2373 = property on="CCD 1D Spectrum Main" class="XYGraph (strict)"("Visible"=w2831) -> ()  [unwired: 2 in, 2 out]
                n2374 = property on="Background substract" class="Enum (strict)"("Visible"=w2830) -> ()  [unwired: 2 in, 2 out]
                n2375 = property on="Accumulations" class="DigNum (strict)"("Visible"=w2830) -> ()  [unwired: 2 in, 2 out]
                n2376 = property on="Exit mirror" class="Ring (strict)"("Val(Sgnl)"=u16 5 ("Value (Signaling)")) -> ()  [unwired: 2 in, 2 out]
                n2377 = property on="CCD ROI" class="Enum (strict)"("Visible"=w2830) -> ()  [unwired: 2 in, 2 out]
                n2378 = property on="CCD 2D Image Main" class="IntGraph (strict)"("Visible"=w2830) -> ()  [unwired: 2 in, 2 out]
                n2379 = property on="CCD 2D Image XY Map" class="IntGraph (strict)"("Visible"=w2830) -> ()  [unwired: 2 in, 2 out]
                n2380 = property on="Exposure Time (ms)" class="DigNum (strict)"("Visible"=w2830) -> ()  [unwired: 2 in, 2 out]
              }
            }
            n2381 = local write "Background taken?"(FALSE ("Background taken?")) -> ()
          }
          event "Acq Time (ms)": Value Change {
            n2382 = event-data() -> ("NewVal"=w2833:dbl)  [unwired: 1 in, 5 out]
            n2383 = local read "Acq Mode"() -> (w2834:T3)
            n2384 = case shown="\"Spectrum\", Default" w2834 {
              tunnel: w2833 -> [w2835 w2836]
              frame "Image" {
                n2385 = property on="Exposure Time (ms)" class="DigNum (strict)"("Val(Sgnl)"=w2835) -> ()  [unwired: 2 in, 2 out]
              }
              frame "Spectrum", Default {
                n2386 = property on="Exposure Time (ms)" class="DigNum (strict)"("Val(Sgnl)"=w2836) -> ()  [unwired: 2 in, 2 out]
              }
            }
            n2387 = local write "Background taken?"(FALSE ("Background taken?")) -> ()
          }
          event "Att Amp", "Att Freq", "Att DCLvl", "ANC Axis": Value Change {
            n2388 = event-data() -> ("CtlRef"=w2844:refnum<vi>)  [unwired: 1 in, 5 out]
            n2389 = local read "Att DeviceHandle"() -> (w2841:u64)
            n2390 = property class="Num"(reference=w2844) -> ("Label.Text"=w2843:string)  [unwired: 1 in, 2 out]
            n2391 = local read "ANC Axis"() -> (w2837:u8)
            n2392 = local read "Att Error"() -> (w2842:errorcluster)
            n2393 = local read "ourDLL"() -> (w2838:path)
            n2394 = case shown="\"ANC Axis\", Default" w2843 {
              tunnel: w2842 -> [w2850 w2856 w2864 w2873]
              tunnel: w2841 -> [w2851 w2857 w2865 w2872]
              tunnel: [w2849 w2855 w2863 w2870] -> w2840
              tunnel: [w2848 w2854 w2862 w2871] -> w2839
              tunnel: w2838 -> [w2847 w2858 w2860 w2869]
              tunnel: w2837 -> [w2845 w2852 w2859 w2866]
              frame "Att Freq" {
                n2395 = local read "Att Freq"() -> (w2846:dbl)
                n2396 = call-poly "ANC350v4_Frequency.vi"("deviceHandle"=w2851, "Path to *.DLL"=w2847, "axis"=w2845, "Frequency [Hz] in"=w2846, "error in"=w2850) -> ("deviceHandle"=w2848:u64, "error ANC350v4_frequency"=w2849:errorcluster)  [unwired: 8 in, 1 out]
              }
              frame "Att Amp" {
                n2397 = local read "Att Amp"() -> (w2853:dbl)
                n2398 = call-poly "ANC350v4_Amplitude.vi"("deviceHandle"=w2857, "Path to *.DLL"=w2858, "axis"=w2852, "amplitude in"=w2853, "error in"=w2856) -> ("deviceHandle"=w2854:u64, "error ANC350v4_Amplitude"=w2855:errorcluster)  [unwired: 8 in, 1 out]
              }
              frame "Att DCLvl" {
                n2399 = local read "Att DCLvl"() -> (w2861:dbl)
                n2400 = call "ANC350v4_SetDCVoltage.vi"("deviceHandle"=w2865, "Path to *.DLL"=w2860, "axis"=w2859, "DC voltage"=w2861, "error in"=w2864) -> ("deviceHandle"=w2862:u64, "error ANC350v4_setDCVoltage"=w2863:errorcluster)  [unwired: 8 in, 1 out]
              }
              frame "ANC Axis", Default {
                n2401 = call "ANC350v4_GetDcVoltage.vi"("deviceHandle"=w2872, "Path to *.DLL"=w2869, "axis"=w2866, "error in"=w2873) -> ("deviceHandle"=w2875:u64, "voltage"=w2874:dbl, "error ANC350v4_getDcVoltage"=w2878:errorcluster)  [unwired: 8 in, 1 out]
                n2402 = local write "Att DCLvl"(w2874) -> ()
                n2403 = call-poly "ANC350v4_Frequency.vi"("deviceHandle"=w2875, "Path to *.DLL"=w2869, "axis"=w2866, "error in"=w2878) -> ("deviceHandle"=w2876:u64, "Frequency [Hz] out"=w2868:dbl, "error ANC350v4_frequency"=w2877:errorcluster)  [unwired: 8 in, 1 out]
                n2404 = local write "Att Freq"(w2868) -> ()
                n2405 = call-poly "ANC350v4_Amplitude.vi"("deviceHandle"=w2876, "Path to *.DLL"=w2869, "axis"=w2866, "error in"=w2877) -> ("deviceHandle"=w2871:u64, "amplitude out"=w2867:dbl, "error ANC350v4_Amplitude"=w2870:errorcluster)  [unwired: 8 in, 1 out]
                n2406 = local write "Att Amp"(w2867) -> ()
              }
            }
            n2407 = local write "Att DeviceHandle"(w2839) -> ()
            n2408 = local write "Att Error"(w2840) -> ()
          }
          event "Att Pos X", "Att Pos Y", "Att Pos Z": Value Change {